vi "Dresden R2R Sputter 03.02.2018 IY24.vi"() -> ()   [LabVIEW 2009] (continued)
                                }
                                frame #1 {
                                }
                                }
                                }
                                frame #1 {
                                n18237 = local read "Semi"() -> (w26574:bool)
                                n18238 = case shown="False" w26574 {
                                frame #0 {
                                n18239 = local write "Ch2_PA31"(TRUE ("PA3")) -> ()
                                n18240 = Wait Until Next ms Multiple(millisecond multiple=u32 1000) -> ()  [unwired: 1 out]
                                }
                                frame #1 {
                                }
                                }
                                }
                                }
                              }
                              frame #1 {
                              }
                            }
                          }
                        }
                      }
                      frame #1 {
                      }
                    }
                  }
                }
              }
              frame #1 {
              }
            }
          }
          frame #2 {
            # "ROUTINE CHECK"
            n18241 = local read "Semi"() -> (w26577:bool)
            n18242 = case shown="False" w26577 {
              frame #0 {
                n18243 = stacked-sequence {
                  frame #0 {
                    n18244 = local read "Semi"() -> (w26578:bool)
                    n18245 = case shown="False" w26578 {
                      frame #0 {
                        n18246 = stacked-sequence {
                          frame #0 {
                            n18247 = local read "Semi"() -> (w26579:bool)
                            n18248 = case shown="False" w26579 {
                              frame #0 {
                                n18249 = while {
                                i -> [w26588]
                                stop <- w26583 stop-if-true
                                n18250 = Greater?(x=w26588, y=400) -> (0:w26586:bool)
                                n18251 = case shown="True" w26586 {
                                frame #0 {
                                }
                                frame #1 {
                                n18252 = local write "Error Message"("Start up process was cancelled.\nPlease check Chamber \nvacuum connections." ("Error Message")) -> ()
                                n18253 = local write "Semi"(TRUE ("Semi")) -> ()
                                }
                                }
                                n18254 = local read "Ch2_pressure"() -> (w26580:dbl)
                                n18255 = Less?(x=w26580, y=0.01) -> (x < y?=w26581:bool)
                                n18256 = case shown="False" w26581 {
                                tunnel: [TRUE FALSE] -> w26585
                                frame #0 {
                                }
                                frame #1 {
                                n18257 = Wait Until Next ms Multiple(millisecond multiple=u32 500) -> ()  [unwired: 1 out]
                                }
                                }
                                n18258 = local read "Semi"() -> (w26584:bool)
                                n18259 = Or(x=w26585, y=w26584) -> (x .or. y?=w26583:bool)
                                }
                              }
                              frame #1 {
                              }
                            }
                          }
                          frame #1 {
                            n18260 = local read "Semi"() -> (w26594:bool)
                            n18261 = case shown="False" w26594 {
                              frame #0 {
                                n18262 = Wait Until Next ms Multiple(millisecond multiple=u32 1000) -> ()  [unwired: 1 out]
                              }
                              frame #1 {
                              }
                            }
                          }
                        }
                      }
                      frame #1 {
                      }
                    }
                  }
                  frame #1 {
                    n18263 = local read "Semi"() -> (w26596:bool)
                    n18264 = case shown="False" w26596 {
                      frame #0 {
                        n18265 = stacked-sequence {
                          frame #0 {
                            n18266 = local read "Semi"() -> (w26597:bool)
                            n18267 = case shown="False" w26597 {
                              frame #0 {
                                n18268 = while {
                                i -> [w26604]
                                stop <- w26598 stop-if-true
                                n18269 = Greater?(x=w26604, y=80) -> (0:w26602:bool)
                                n18270 = case shown="True" w26602 {
                                frame #0 {
                                }
                                frame #1 {
                                n18271 = local write "Semi"(TRUE ("Semi")) -> ()
                                n18272 = local write "Error Message"("Start up process  cancelled\nbecause  CC not opened.\nPlease check CH2-CC connections." ("Error Message")) -> ()
                                }
                                }
                                n18273 = local read "Ch2_Cc_on_off_di"() -> (w26601:bool)
                                n18274 = case shown="False" w26601 {
                                tunnel: [TRUE FALSE] -> w26600
                                frame #0 {
                                }
                                frame #1 {
                                n18275 = Wait Until Next ms Multiple(millisecond multiple=u32 200) -> ()  [unwired: 1 out]
                                n18276 = local write "Ch2_Cc_on_off_do"(TRUE ("Ch1_Tp_bv_do")) -> ()
                                }
                                }
                                n18277 = local read "Semi"() -> (w26599:bool)
                                n18278 = Or(x=w26600, y=w26599) -> (x .or. y?=w26598:bool)
                                }
                              }
                              frame #1 {
                              }
                            }
                          }
                          frame #1 {
                            n18279 = local read "Semi"() -> (w26611:bool)
                            n18280 = case shown="False" w26611 {
                              frame #0 {
                                n18281 = while {
                                i -> [w26615]
                                stop <- w26612 stop-if-true
                                n18282 = Greater Or Equal?(x=w26615, y=150) -> (x >= y?=w26613:bool)
                                n18283 = Wait (ms)(milliseconds to wait=u32 200) -> ()  [unwired: 1 out]
                                n18284 = local read "Semi"() -> (w26617:bool)
                                n18285 = Compound Arithmetic op=OR(w26613, w26617) -> (w26612:bool)
                                }
                              }
                              frame #1 {
                              }
                            }
                          }
                          frame #2 {
                            n18286 = local read "Semi"() -> (w26618:bool)
                            n18287 = case shown="False" w26618 {
                              frame #0 {
                                n18288 = local write "Ch2_PA32"(TRUE ("P1")) -> ()
                                n18289 = local write "Ch2_PV21"(TRUE ("P1")) -> ()
                                n18290 = Wait Until Next ms Multiple(millisecond multiple=u32 2000) -> ()  [unwired: 1 out]
                              }
                              frame #1 {
                              }
                            }
                          }
                        }
                      }
                      frame #1 {
                      }
                    }
                  }
                  frame #2 {
                    n18291 = local read "Semi"() -> (w26622:bool)
                    n18292 = case shown="False" w26622 {
                      frame #0 {
                        n18293 = stacked-sequence {
                          frame #0 {
                            n18294 = local read "Semi"() -> (w26623:bool)
                            n18295 = case shown="False" w26623 {
                              frame #0 {
                                n18296 = while {
                                i -> [w26630]
                                stop <- w26624 stop-if-true
                                n18297 = Greater?(x=w26630, y=80) -> (0:w26628:bool)
                                n18298 = case shown="True" w26628 {
                                frame #0 {
                                }
                                frame #1 {
                                n18299 = local write "Semi"(TRUE ("Semi")) -> ()
                                n18300 = local write "Error Message"("Start up process  cancelled\nbecause  CH2-TRNS-GV-BP\n not opened.\nPlease check CH2-TRNS-GV-BP\n connections." ("Error Message")) -> ()
                                }
                                }
                                n18301 = local read "Ch2_trns_gv_bp_di"() -> (w26627:bool)
                                n18302 = case shown="True" w26627 {
                                tunnel: [FALSE TRUE] -> w26626
                                frame #0 {
                                n18303 = Wait Until Next ms Multiple(millisecond multiple=u32 200) -> ()  [unwired: 1 out]
                                n18304 = local write "Ch2_trns_gv_bp_do"(FALSE ("Ch1_Tp_bv_do")) -> ()
                                }
                                frame #1 {
                                }
                                }
                                n18305 = local read "Semi"() -> (w26625:bool)
                                n18306 = Or(x=w26626, y=w26625) -> (x .or. y?=w26624:bool)
                                }
                              }
                              frame #1 {
                              }
                            }
                          }
                          frame #1 {
                            n18307 = local read "Semi"() -> (w26637:bool)
                            n18308 = case shown="False" w26637 {
                              frame #0 {
                                n18309 = local write "Ch2_PA33"(TRUE ("P1")) -> ()
                                n18310 = local write "Ch2_PV22"(TRUE ("P1")) -> ()
                                n18311 = Wait Until Next ms Multiple(millisecond multiple=u32 2000) -> ()  [unwired: 1 out]
                              }
                              frame #1 {
                              }
                            }
                          }
                        }
                      }
                      frame #1 {
                      }
                    }
                  }
                  frame #3 {
                    n18312 = local read "Semi"() -> (w26641:bool)
                    n18313 = case shown="False" w26641 {
                      frame #0 {
                        n18314 = stacked-sequence {
                          frame #0 {
                            n18315 = local read "Semi"() -> (w26642:bool)
                            n18316 = case shown="False" w26642 {
                              frame #0 {
                                n18317 = while {
                                i -> [w26649]
                                stop <- w26643 stop-if-true
                                n18318 = Greater?(x=w26649, y=80) -> (0:w26647:bool)
                                n18319 = case shown="True" w26647 {
                                frame #0 {
                                }
                                frame #1 {
                                n18320 = local write "Semi"(TRUE ("Semi")) -> ()
                                n18321 = local write "Error Message"("Start up process  cancelled\nbecause  CH2-TRNS-GV-BP2\n not opened.\nPlease check CH2-TRNS-GV-BP2\n connections." ("Error Message")) -> ()
                                }
                                }
                                n18322 = local read "Ch2_trns_gv_bp2_di"() -> (w26646:bool)
                                n18323 = case shown="True" w26646 {
                                tunnel: [FALSE TRUE] -> w26645
                                frame #0 {
                                n18324 = local write "Ch2_trns_gv_bp2_do"(FALSE ("Ch1_Tp_bv_do")) -> ()
                                n18325 = Wait Until Next ms Multiple(millisecond multiple=u32 200) -> ()  [unwired: 1 out]
                                }
                                frame #1 {
                                }
                                }
                                n18326 = local read "Semi"() -> (w26644:bool)
                                n18327 = Or(x=w26645, y=w26644) -> (x .or. y?=w26643:bool)
                                }
                              }
                              frame #1 {
                              }
                            }
                          }
                          frame #1 {
                            n18328 = local read "Semi"() -> (w26656:bool)
                            n18329 = case shown="False" w26656 {
                              frame #0 {
                                n18330 = local write "Ch2_PA34"(TRUE ("P1")) -> ()
                                n18331 = local write "Ch2_PV23"(TRUE ("P1")) -> ()
                                n18332 = Wait Until Next ms Multiple(millisecond multiple=u32 2000) -> ()  [unwired: 1 out]
                              }
                              frame #1 {
                              }
                            }
                          }
                        }
                      }
                      frame #1 {
                      }
                    }
                  }
                  frame #4 {
                    n18333 = local read "Semi"() -> (w26660:bool)
                    n18334 = case shown="False" w26660 {
                      frame #0 {
                        n18335 = stacked-sequence {
                          frame #0 {
                            n18336 = local read "Semi"() -> (w26661:bool)
                            n18337 = case shown="False" w26661 {
                              frame #0 {
                                n18338 = while {
                                i -> [w26670]
                                stop <- w26665 stop-if-true
                                n18339 = local read "Target_time_ch2"() -> (w26664:dbl)
                                n18340 = Multiply(x=w26664, y=7200) -> (x*y=w26662:dbl)
                                n18341 = Greater?(x=w26670, y=w26662) -> (0:w26669:bool)
                                n18342 = case shown="True" w26669 {
                                frame #0 {
                                }
                                frame #1 {
                                n18343 = local write "Semi"(TRUE ("Semi")) -> ()
                                }
                                }
                                n18344 = local read "Semi"() -> (w26668:bool)
                                n18345 = case shown="False" w26668 {
                                tunnel: [TRUE w26675] -> w26667
                                frame #0 {
                                }
                                frame #1 {
                                n18346 = local read "Target Pressure_ch2"() -> (w26674:dbl)
                                n18347 = local read "Ch2_pressure"() -> (w26673:dbl)
                                n18348 = Less Or Equal?(x=w26674, y=w26673) -> (x <= y?=w26672:bool)
                                n18349 = case shown="True" w26672 {
                                tunnel: [TRUE FALSE] -> w26675
                                frame #0 {
                                }
                                frame #1 {
                                n18350 = Wait Until Next ms Multiple(millisecond multiple=u32 750) -> ()  [unwired: 1 out]
                                }
                                }
                                }
                                }
                                n18351 = local read "Semi"() -> (w26666:bool)
                                n18352 = Or(x=w26667, y=w26666) -> (x .or. y?=w26665:bool)
                                }
                              }
                              frame #1 {
                              }
                            }
                          }
                          frame #1 {
                            n18353 = local read "Semi"() -> (w26680:bool)
                            n18354 = case shown="False" w26680 {
                              frame #0 {
                                n18355 = Wait (ms)(milliseconds to wait=u32 1000) -> ()  [unwired: 1 out]
                              }
                              frame #1 {
                              }
                            }
                          }
                          frame #2 {
                            n18356 = local read "Semi"() -> (w26682:bool)
                            n18357 = case shown="False" w26682 {
                              frame #0 {
                                n18358 = local write "Ch2_PA35"(TRUE ("P1")) -> ()
                                n18359 = local write "Ch2_PV24"(TRUE ("P1")) -> ()
                                n18360 = Wait Until Next ms Multiple(millisecond multiple=u32 1000) -> ()  [unwired: 1 out]
                              }
                              frame #1 {
                              }
                            }
                          }
                        }
                      }
                      frame #1 {
                      }
                    }
                  }
                }
              }
              frame #1 {
              }
            }
          }
          frame #3 {
            # "ROUTINE CHECK"
            n18361 = local read "Semi"() -> (w26686:bool)
            n18362 = case shown="False" w26686 {
              frame #0 {
                n18363 = stacked-sequence {
                  frame #0 {
                    n18364 = local read "Semi"() -> (w26687:bool)
                    n18365 = case shown="False" w26687 {
                      frame #0 {
                        w26688 = TRUE ("Visible")
                        n18366 = local write "system_status"("Start up was completed." ("system_status")) -> ()
                        n18367 = property on="final_mes_tab" class="TabCtl (strict)"("Visible"=w26688) -> ()  [unwired: 2 in, 2 out]
                        n18368 = local write "Cnt_Do_Buzzer"(w26688) -> ()
                        n18369 = Wait (ms)(milliseconds to wait=u32 3000 ("millisecond multiple")) -> ()  [unwired: 1 out]
                      }
                      frame #1 {
                      }
                    }
                  }
                  frame #1 {
                    n18370 = local read "Semi"() -> (w26691:bool)
                    n18371 = case shown="False" w26691 {
                      frame #0 {
                        w26692 = FALSE ("Visible")
                        n18372 = local write "system_status"("" ("system_status")) -> ()
                        n18373 = local write "Cnt_Do_Buzzer"(w26692) -> ()
                        n18374 = Wait (ms)(milliseconds to wait=u32 3000 ("millisecond multiple")) -> ()  [unwired: 1 out]
                        n18375 = property on="final_mes_tab" class="TabCtl (strict)"("Visible"=w26692) -> ()  [unwired: 2 in, 2 out]
                        n18376 = local write "Start_up_ch2"(w26692) -> ()
                      }
                      frame #1 {
                      }
                    }
                  }
                  frame #2 {
                    n18377 = local read "Semi"() -> (w26695:bool)
                    n18378 = case shown="False" w26695 {
                      frame #0 {
                        n18379 = stacked-sequence {
                          frame #0 {
                            n18380 = local write "Pps_code_entry"("PF331=" ("system_status")) -> ()
                          }
                          frame #1 {
                            n18381 = Wait (ms)(milliseconds to wait=u32 500) -> ()  [unwired: 1 out]
                          }
                          frame #2 {
                            n18382 = local write "Ppsok"(TRUE ("Ppsok")) -> ()
                          }
                          frame #3 {
                            n18383 = Wait (ms)(milliseconds to wait=u32 1000) -> ()  [unwired: 1 out]
                          }
                        }
                      }
                      frame #1 {
                      }
                    }
                  }
                  frame #3 {
                    n18384 = local read "Semi"() -> (w26700:bool)
                    n18385 = case shown="False" w26700 {
                      frame #0 {
                        n18386 = stacked-sequence {
                          frame #0 {
                            n18387 = local write "Pps_code_entry"("PF227=" ("system_status")) -> ()
                          }
                          frame #1 {
                            n18388 = Wait (ms)(milliseconds to wait=u32 500) -> ()  [unwired: 1 out]
                          }
                          frame #2 {
                            n18389 = local write "Ppsok"(TRUE ("Ppsok")) -> ()
                          }
                          frame #3 {
                            n18390 = Wait (ms)(milliseconds to wait=u32 1000) -> ()  [unwired: 1 out]
                          }
                        }
                      }
                      frame #1 {
                      }
                    }
                  }
                  frame #4 {
                    n18391 = local read "Semi"() -> (w26705:bool)
                    n18392 = case shown="False" w26705 {
                      frame #0 {
                        n18393 = stacked-sequence {
                          frame #0 {
                            n18394 = local write "Pps_code_entry"("PF330=" ("system_status")) -> ()
                          }
                          frame #1 {
                            n18395 = Wait (ms)(milliseconds to wait=u32 500) -> ()  [unwired: 1 out]
                          }
                          frame #2 {
                            n18396 = local write "Ppsok"(TRUE ("Ppsok")) -> ()
                          }
                          frame #3 {
                            n18397 = Wait (ms)(milliseconds to wait=u32 1000) -> ()  [unwired: 1 out]
                          }
                        }
                      }
                      frame #1 {
                      }
                    }
                  }
                  frame #5 {
                    n18398 = local read "Semi"() -> (w26710:bool)
                    n18399 = case shown="False" w26710 {
                      frame #0 {
                        w26711 = FALSE ("PB34")
                        n18400 = local write "Ch2_PV25"(w26711) -> ()
                        n18401 = local write "Ch2_PA36"(w26711) -> ()
                        n18402 = Wait (ms)(milliseconds to wait=u32 1000) -> ()  [unwired: 1 out]
                      }
                      frame #1 {
                      }
                    }
                  }
                }
              }
              frame #1 {
              }
            }
          }
        }
      }
    }
    n18403 = case shown="True" "Shutdown_ch2" {
      frame #0 {
      }
      frame #1 {
        n18404 = local read "Semi"() -> (w24982:bool)
        n18405 = case shown="False" w24982 {
          frame #0 {
            n18406 = stacked-sequence {
              frame #0 {
                n18407 = local read "Semi"() -> (w24983:bool)
                n18408 = case shown="False" w24983 {
                  frame #0 {
                    n18409 = stacked-sequence {
                      frame #0 {
                        w24986 = FALSE
                        n18410 = local write "final_process_messages"("Shut Down process was completed." ("final_process_messages")) -> ()
                        n18411 = local write "system_status"("Shutting Down the System" ("system_status")) -> ()
                        n18412 = local write "Clean_shutdown_ch2"(TRUE) -> ()
                        n18413 = Wait (ms)(milliseconds to wait=u32 1000) -> ()  [unwired: 1 out]
                        "Yes 2" <- w24986
                        "No 2" <- w24986
                        "Cancel 2" <- w24986
                        "Close 2" <- w24986
                      }
                      frame #1 {
                        n18414 = call <vilib>:"Three Button Dialog.vi"("Right Button Text (\"Cancel\")"="Cancel" ("Right Button Text (\"Cancel\")"), "Center Button Text (\"No\")"="No" ("Center Button Text (\"No\")"), "Left Button Text (\"Yes\")"="Yes" ("Left Button Text (\"Yes\")"), "message"=" VENT the CHAMBER  \nLOAD or UNLOAD the substrate ? ") -> ("Which Button?"=w24992:T40)  [unwired: 7 in]
                        n18415 = case shown="\"Window Close\"" w24992 {
                          frame #0 {
                            n18416 = local write "Yes 2"(TRUE ("Close")) -> ()
                          }
                          frame #1 {
                            n18417 = local write "Close 2"(TRUE ("Close")) -> ()
                          }
                          frame #2 {
                            n18418 = local write "Cancel 2"(TRUE ("No")) -> ()
                          }
                          frame #3 {
                            n18419 = local write "No 2"(TRUE ("No")) -> ()
                          }
                        }
                      }
                      frame #2 {
                        n18420 = local read "Semi"() -> (w24998:bool)
                        n18421 = case shown="False" w24998 {
                          frame #0 {
                            n18422 = stacked-sequence {
                              frame #0 {
                                n18423 = local write "Error Message"("" ("Error Message")) -> ()
                              }
                              frame #1 {
                                n18424 = Wait (ms)(milliseconds to wait=u32 500) -> ()  [unwired: 1 out]
                              }
                              frame #2 {
                                n18425 = local write "Ppsok"(TRUE ("Ppsok")) -> ()
                              }
                              frame #3 {
                                n18426 = Wait (ms)(milliseconds to wait=u32 500) -> ()  [unwired: 1 out]
                              }
                            }
                          }
                          frame #1 {
                          }
                        }
                      }
                    }
                  }
                  frame #1 {
                  }
                }
              }
              frame #1 {
                n18427 = local read "Semi"() -> (w25003:bool)
                n18428 = case shown="False" w25003 {
                  frame #0 {
                    n18429 = local read "Cancel 2"() -> (w25005:bool)
                    n18430 = local read "Close 2"() -> (w25006:bool)
                    n18431 = Not Or(1:w25005, 2:w25006) -> (0:w25004:bool)
                    n18432 = case shown="True" w25004 {
                      frame #0 {
                        n18433 = local read "Semi"() -> (w25007:bool)
                        n18434 = case shown="False" w25007 {
                          frame #0 {
                          }
                          frame #1 {
                            n18435 = local write "system_status"("Semi-automatic is active" ("system_status")) -> ()
                            n18436 = local write "Shutdown_ch2"(FALSE ("Shutdown_ch1")) -> ()
                          }
                        }
                      }
                      frame #1 {
                        n18437 = local read "Yes 2"() -> (w25012:bool)
                        n18438 = local read "No 2"() -> (w25011:bool)
                        n18439 = Or(x=w25012, y=w25011) -> (x .or. y?=w25010:bool)
                        n18440 = case shown="True" w25010 {
                          frame #0 {
                          }
                          frame #1 {
                            n18441 = stacked-sequence {
                              frame #0 {
                                # "CLOSE & ZERO ROUTINES"
                                n18442 = local read "Semi"() -> (w25013:bool)
                                n18443 = case shown="False" w25013 {
                                frame #0 {
                                n18444 = stacked-sequence {
                                frame #0 {
                                n18445 = local read "Semi"() -> (w25014:bool)
                                n18446 = case shown="False" w25014 {
                                frame #0 {
                                w25016 = TRUE ("Dc_auto_off")
                                n18447 = local write "Dc_auto_off"(w25016) -> ()
                                n18448 = local write "Ar_auto_set_zero_ch2"(w25016) -> ()
                                n18449 = local write "system_status"("Shut Down in Progress for Chamber 2" ("system_status")) -> ()
                                n18450 = local write "final_process_messages"("Shut Down Process was completed for  Chamber 2." ("final_process_messages")) -> ()
                                n18451 = local write "Ch2_Sov_Ar_do"(FALSE ("Dc_auto_off")) -> ()
                                }
                                frame #1 {
                                }
                                }
                                }
                                frame #1 {
                                n18452 = local read "Semi"() -> (w25019:bool)
                                n18453 = case shown="False" w25019 {
                                frame #0 {
                                n18454 = Wait (ms)(milliseconds to wait=u32 2500) -> ()  [unwired: 1 out]
                                }
                                frame #1 {
                                }
                                }
                                }
                                frame #2 {
                                n18455 = local read "Semi"() -> (w25021:bool)
                                n18456 = case shown="False" w25021 {
                                frame #0 {
                                n18457 = local write "Ch2_Sov_Ar_do"(FALSE ("Ch1_Sov_Ar_do")) -> ()
                                n18458 = Wait (ms)(milliseconds to wait=u32 2500) -> ()  [unwired: 1 out]
                                n18459 = local write "RF_auto_off"(TRUE ("RF_auto_off")) -> ()
                                }
                                frame #1 {
                                }
                                }
                                }
                                frame #3 {
                                n18460 = local read "Semi"() -> (w25025:bool)
                                n18461 = case shown="False" w25025 {
                                frame #0 {
                                n18462 = Wait (ms)(milliseconds to wait=u32 1000) -> ()  [unwired: 1 out]
                                }
                                frame #1 {
                                }
                                }
                                }
                                }
                                }
                                frame #1 {
                                }
                                }
                              }
                              frame #1 {
                                # "STOP TP"
                                n18463 = local read "Semi"() -> (w25027:bool)
                                n18464 = case shown="False" w25027 {
                                frame #0 {
                                n18465 = stacked-sequence {
                                frame #0 {
                                n18466 = local read "Semi"() -> (w25028:bool)
                                n18467 = case shown="False" w25028 {
                                frame #0 {
                                n18468 = stacked-sequence {
                                frame #0 {
                                n18469 = local read "Semi"() -> (w25029:bool)
                                n18470 = case shown="False" w25029 {
                                frame #0 {
                                n18471 = local write "Tp2_auto_stop"(TRUE ("Tp1_auto_start")) -> ()
                                }
                                frame #1 {
                                }
                                }
                                }
                                frame #1 {
                                n18472 = local read "Semi"() -> (w25031:bool)
                                n18473 = case shown="False" w25031 {
                                frame #0 {
                                n18474 = Wait (ms)(milliseconds to wait=u32 1000) -> ()  [unwired: 1 out]
                                }
                                frame #1 {
                                }
                                }
                                }
                                frame #2 {
                                n18475 = local read "Semi"() -> (w25033:bool)
                                n18476 = case shown="False" w25033 {
                                frame #0 {
                                n18477 = while {
                                i -> [w25039]
                                stop <- w25035 stop-if-true
                                n18478 = local read "Tp2_stopped"() -> (w25037:bool)
                                n18479 = Greater?(x=w25039, y=120) -> (0:w25038:bool)
                                n18480 = local read "Semi"() -> (w25036:bool)
                                n18481 = Compound Arithmetic op=OR(w25036, w25037, w25038) -> (w25035:bool)
                                n18482 = Wait (ms)(milliseconds to wait=u32 500) -> ()  [unwired: 1 out]
                                }
                                }
                                frame #1 {
                                }
                                }
                                }
                                frame #3 {
                                n18483 = local read "Semi"() -> (w25041:bool)
                                n18484 = case shown="False" w25041 {
                                frame #0 {
                                n18485 = local read "Tp2_stopped"() -> (w25042:bool)
                                n18486 = case shown="False" w25042 {
                                frame #0 {
                                n18487 = local write "Tp2_auto_stop"(TRUE ("Pc_bv1_auto_open")) -> ()
                                }
                                frame #1 {
                                }
                                }
                                }
                                frame #1 {
                                }
                                }
                                }
                                frame #4 {
                                n18488 = local read "Semi"() -> (w25044:bool)
                                n18489 = case shown="False" w25044 {
                                frame #0 {
                                n18490 = local read "Tp2_stopped"() -> (w25045:bool)
                                n18491 = case shown="False" w25045 {
                                frame #0 {
                                n18492 = Wait (ms)(milliseconds to wait=u32 1000) -> ()  [unwired: 1 out]
                                }
                                frame #1 {
                                }
                                }
                                }
                                frame #1 {
                                }
                                }
                                }
                                frame #5 {
                                n18493 = local read "Semi"() -> (w25047:bool)
                                n18494 = case shown="False" w25047 {
                                frame #0 {
                                n18495 = while {
                                i -> [w25053]
                                stop <- w25049 stop-if-true
                                n18496 = local read "Tp2_stopped"() -> (w25051:bool)
                                n18497 = Greater?(x=w25053, y=120) -> (0:w25052:bool)
                                n18498 = local read "Semi"() -> (w25050:bool)
                                n18499 = Compound Arithmetic op=OR(w25050, w25051, w25052) -> (w25049:bool)
                                n18500 = Wait (ms)(milliseconds to wait=u32 500) -> ()  [unwired: 1 out]
                                }
                                }
                                frame #1 {
                                }
                                }
                                }
                                frame #6 {
                                n18501 = local read "Semi"() -> (w25055:bool)
                                n18502 = case shown="False" w25055 {
                                frame #0 {
                                n18503 = local read "Tp2_stopped"() -> (w25056:bool)
                                n18504 = case shown="False" w25056 {
                                frame #0 {
                                n18505 = local write "Error Message"("Shut Down process  cancelled\nbecause  TP not stopped.\nPlease check TP2 connections." ("Error Message")) -> ()
                                n18506 = local write "Semi"(TRUE ("Semi")) -> ()
                                }
                                frame #1 {
                                }
                                }
                                }
                                frame #1 {
                                }
                                }
                                }
                                }
                                }
                                frame #1 {
                                }
                                }
                                }
                                frame #1 {
                                n18507 = local read "Semi"() -> (w25059:bool)
                                n18508 = case shown="False" w25059 {
                                frame #0 {
                                n18509 = local write "Ch2_Sd1"(TRUE ("Ch1_Sd0")) -> ()
                                n18510 = Wait (ms)(milliseconds to wait=u32 1000) -> ()  [unwired: 1 out]
                                }
                                frame #1 {
                                }
                                }
                                }
                                }
                                }
                                frame #1 {
                                }
                                }
                              }
                              frame #2 {
                                # "CLOSE CC"
                                n18511 = local read "Semi"() -> (w25062:bool)
                                n18512 = case shown="False" w25062 {
                                frame #0 {
                                n18513 = stacked-sequence {
                                frame #0 {
                                n18514 = local read "Semi"() -> (w25063:bool)
                                n18515 = case shown="False" w25063 {
                                frame #0 {
                                n18516 = while {
                                i -> [w25069]
                                stop <- w25064 stop-if-true
                                n18517 = Greater?(x=w25069, y=25) -> (0:w25068:bool)
                                n18518 = case shown="True" w25068 {
                                frame #0 {
                                }
                                frame #1 {
                                n18519 = local write "Error Message"("Shut Down Process  cancelled\nbecause  CC not closed.\nPlease check CH2-CC connections." ("Error Message")) -> ()
                                n18520 = local write "Semi"(TRUE ("Semi")) -> ()
                                }
                                }
                                n18521 = local read "Ch2_Cc_on_off_di"() -> (w25067:bool)
                                n18522 = case shown="True" w25067 {
                                tunnel: [TRUE FALSE] -> w25065
                                frame #0 {
                                }
                                frame #1 {
                                n18523 = local write "Ch2_Cc_on_off_do"(FALSE ("Ch1_Ch_cc_on_off_di")) -> ()
                                n18524 = Wait Until Next ms Multiple(millisecond multiple=u32 200) -> ()  [unwired: 1 out]
                                }
                                }
                                n18525 = local read "Semi"() -> (w25066:bool)
                                n18526 = Or(x=w25065, y=w25066) -> (x .or. y?=w25064:bool)
                                }
                                }
                                frame #1 {
                                }
                                }
                                }
                                frame #1 {
                                n18527 = local read "Semi"() -> (w25077:bool)
                                n18528 = case shown="False" w25077 {
                                frame #0 {
                                n18529 = local write "Ch2_Sd2"(TRUE ("Ch1_Sd1")) -> ()
                                n18530 = Wait (ms)(milliseconds to wait=u32 1000) -> ()  [unwired: 1 out]
                                }
                                frame #1 {
                                }
                                }
                                }
                                }
                                }
                                frame #1 {
                                }
                                }
                              }
                              frame #3 {
                                # "CLOSE BG-BV"
                                n18531 = local read "Semi"() -> (w25080:bool)
                                n18532 = case shown="False" w25080 {
                                frame #0 {
                                n18533 = stacked-sequence {
                                frame #0 {
                                n18534 = local read "Semi"() -> (w25081:bool)
                                n18535 = case shown="False" w25081 {
                                frame #0 {
                                n18536 = while {
                                i -> [w25087]
                                stop <- w25082 stop-if-true
                                n18537 = Greater?(x=w25087, y=25) -> (0:w25086:bool)
                                n18538 = case shown="True" w25086 {
                                frame #0 {
                                }
                                frame #1 {
                                n18539 = local write "Error Message"("Shut Down Process  cancelled\nbecause  BG-BV not closed.\nPlease check BG-BV2 connections." ("Error Message")) -> ()
                                n18540 = local write "Semi"(TRUE ("Semi")) -> ()
                                }
                                }
                                n18541 = local read "Ch2_Bg_bv_di"() -> (w25085:bool)
                                n18542 = case shown="True" w25085 {
                                tunnel: [TRUE FALSE] -> w25083
                                frame #0 {
                                }
                                frame #1 {
                                n18543 = Wait Until Next ms Multiple(millisecond multiple=u32 200) -> ()  [unwired: 1 out]
                                n18544 = local write "Ch2_Bg_bv_do"(FALSE ("Ch1_Ch_cc_on_off_di")) -> ()